vi "A170316-11-Main-large.vi"() -> ()   [LabVIEW 2020]
uses:
  System.Windows.Forms
  Database/Global1.vi
  Global_Variable/A170316-11.vi
  Global_Variable/Global.vi
  <userlib>/_MGI/Menu Building/MenuItemStatusChange/MGI_MenuItemStatusChange.lvclass
panel:
  out "提示信息 2":string
  out "ECU前序显示字":string
  out "电机前序显示字":string
  out "ECU装配\n前序状态":bool
  out "电机装配\n前序状态":bool
  out "电机码":string
  out "电机工位管柱码":string
  out "控制器码":string
  out "ECU自动":bool
  out "电机安装数量":u32
  out "ECU结果显示":string
  out "电机结果显示":string
  in  "质量报警":bool caption="布尔"
  in  "设备缺料":bool caption="布尔"
  in  "设备故障":bool caption="布尔"
  in  "设备离线":bool caption="布尔"
  in  "设备正常":bool caption="布尔"
  in  "菜单":refnum<k24>(container)
  out "检测结果":bool
  in  "批次信息":string[][](table)
  out "提示信息":string
  out "错误":bool
  out "时间字符串":string
  out "日期字符串":string
  out "电机自动":bool
  out "userStatus":string caption="用户状态"
  out "userName":string caption="用户名"
  out "安装支架数量":u32
  out "ECU工位管柱码":string
  out "connectionMode":string caption="联机类型"
  out "产品型号":string
  in  "更换产品":refnum<vi>
  # "电机ECU装配"
  # "控制器支架"
  # "安装支架(合装)"
  # "电机安装"
  # "安装支架检测结果"
  # "电机安装检测结果"
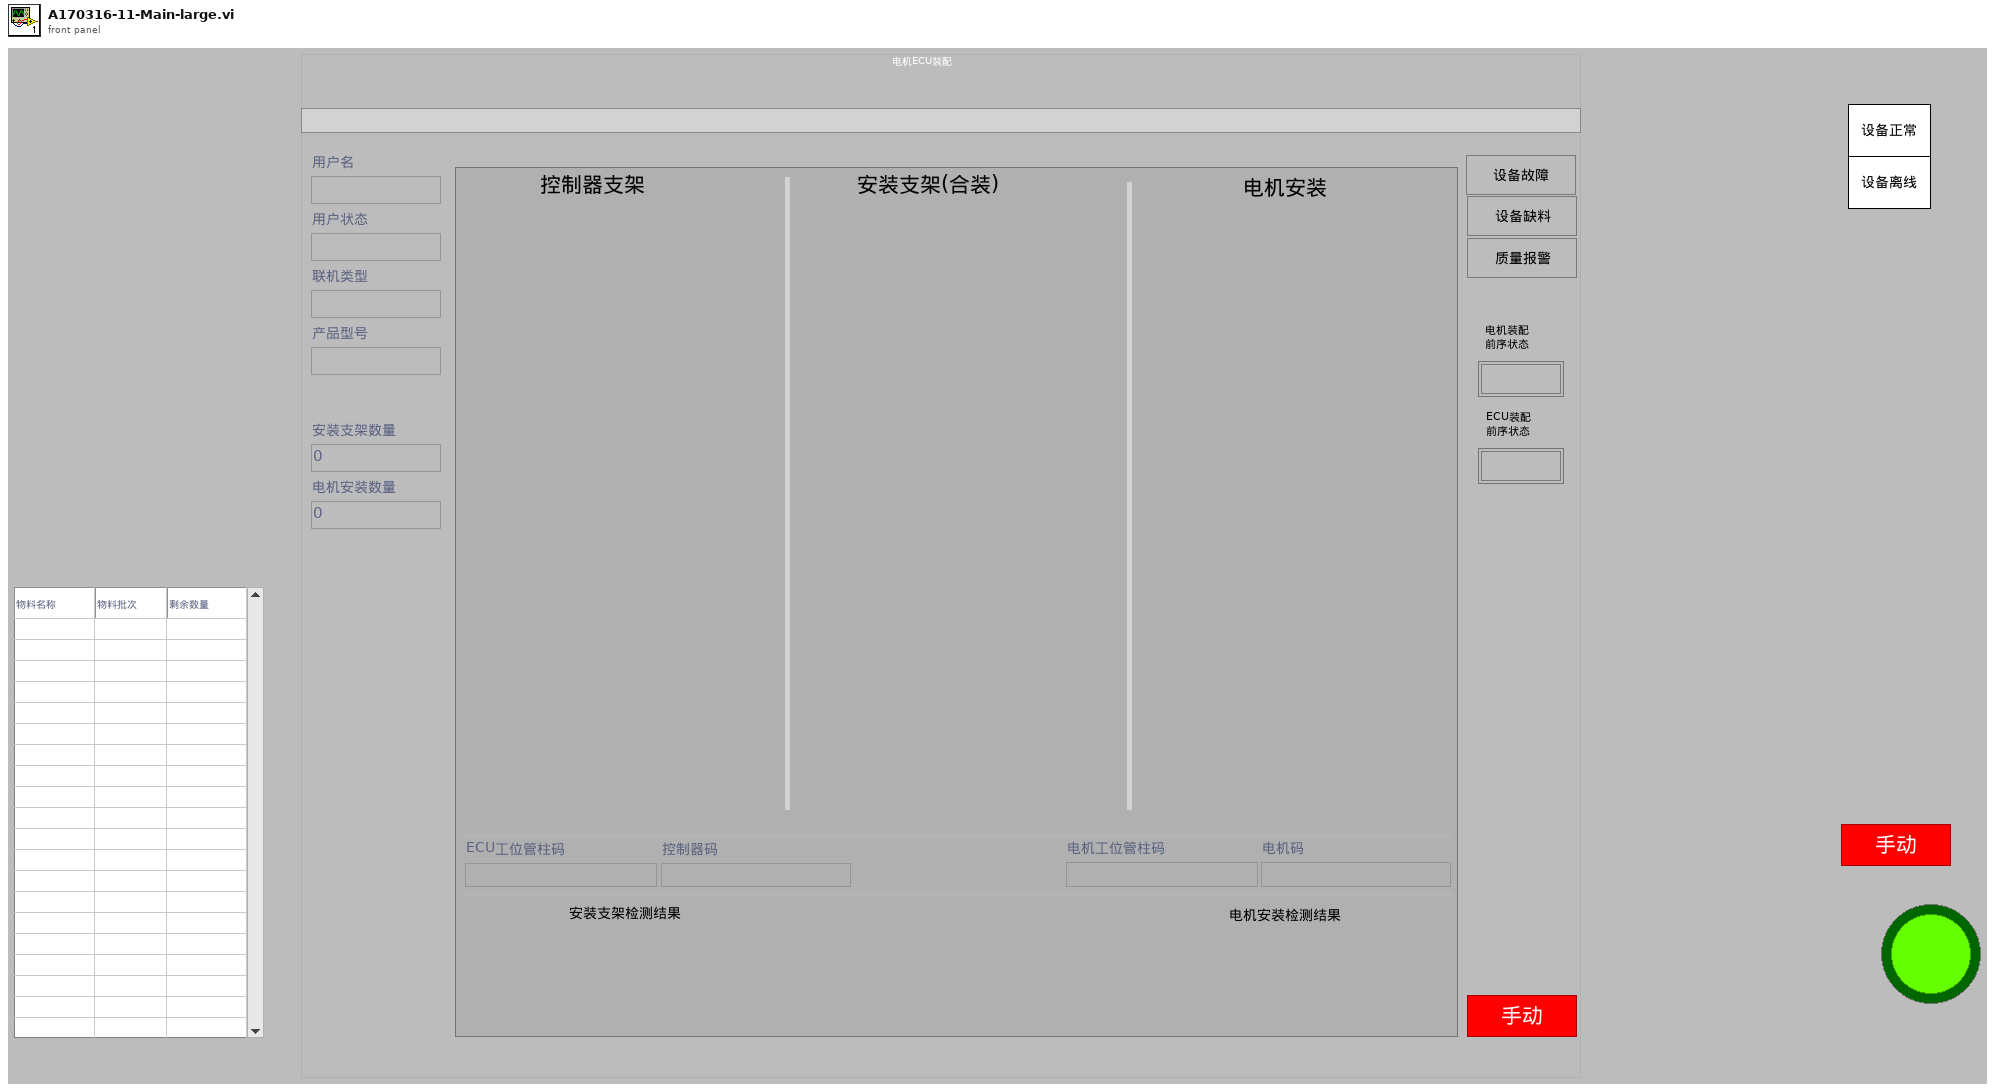
[diagram p1: front panel]
types:
  T1 = enum32{"Invalid", "Standard", "Closed", "Hidden", "Minimized", "Maximized"}
  T2 = enum32{"invalid app kind", "Development System", "Run Time System", "Student Edition", "Embedded LabVIEW", "Evaluation", "Custom"}
  T3 = cluster{"Core":cluster{"Current VI Reference":refnum<vi>, "Close Panel on Exit?":bool}, "Your Boolean data":bool, "Your string data":string}
  T4 = cluster{"Current VI Reference":refnum<vi>, "Close Panel on Exit?":bool}
  T5 = cluster{"用户编号":string, "用户名":string, "用户密码(密文)":string, "用户权限":string}
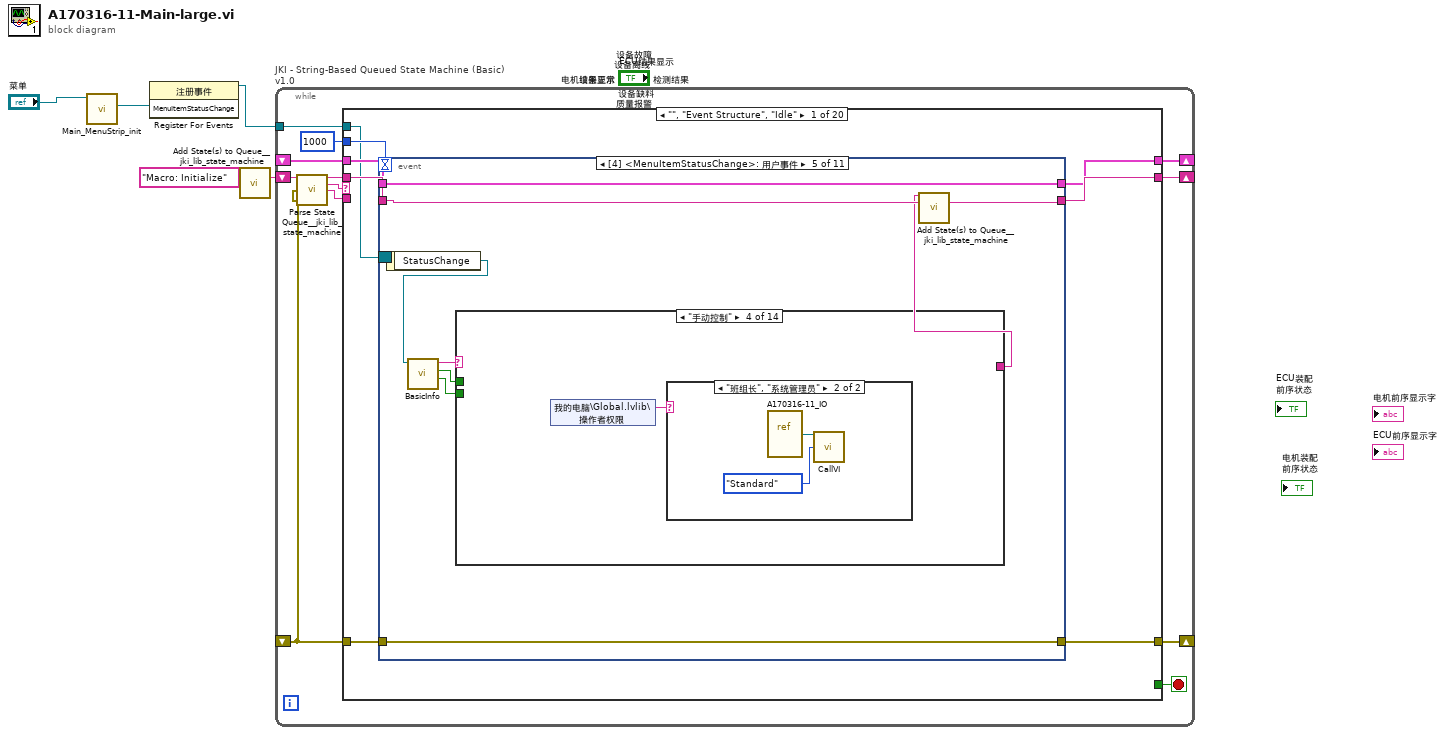
[diagram p0: block diagram]
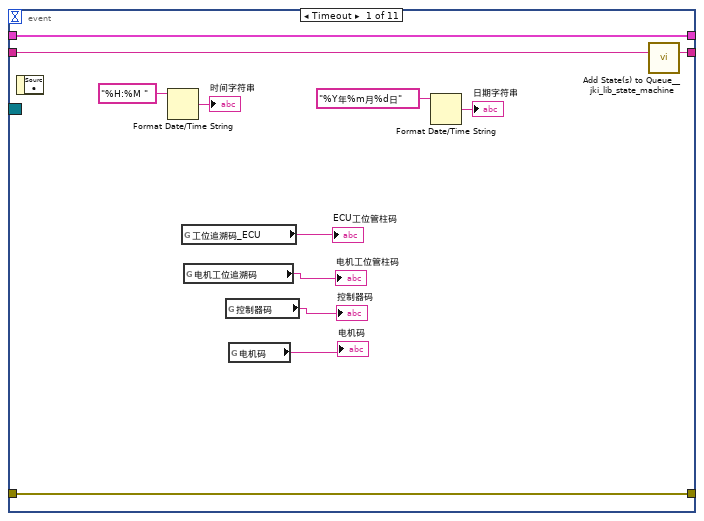
[diagram p2: hidden frame]
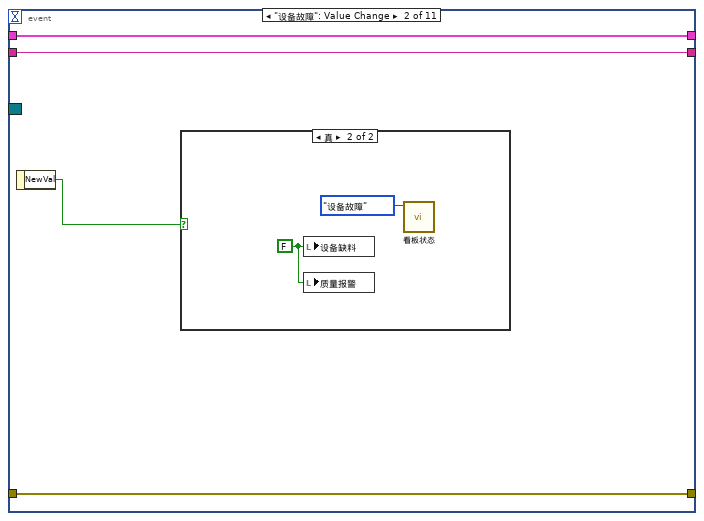
[diagram p3: hidden frame]
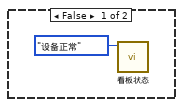
[diagram p4: hidden frame]
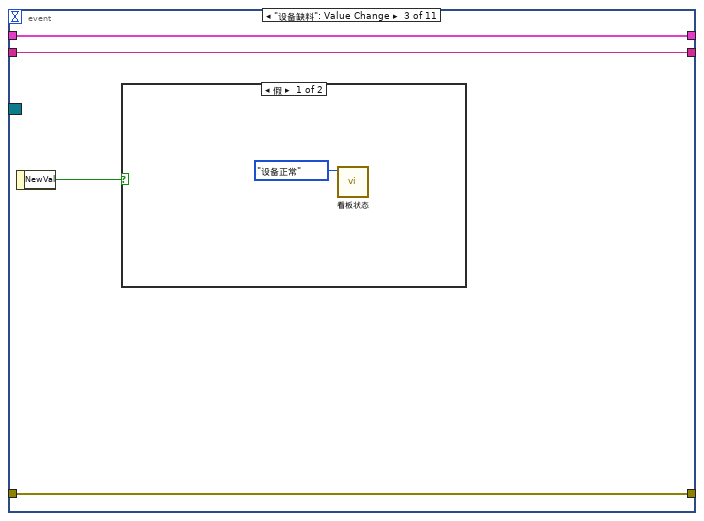
[diagram p5: hidden frame]
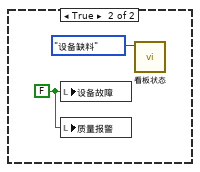
[diagram p6: hidden frame]
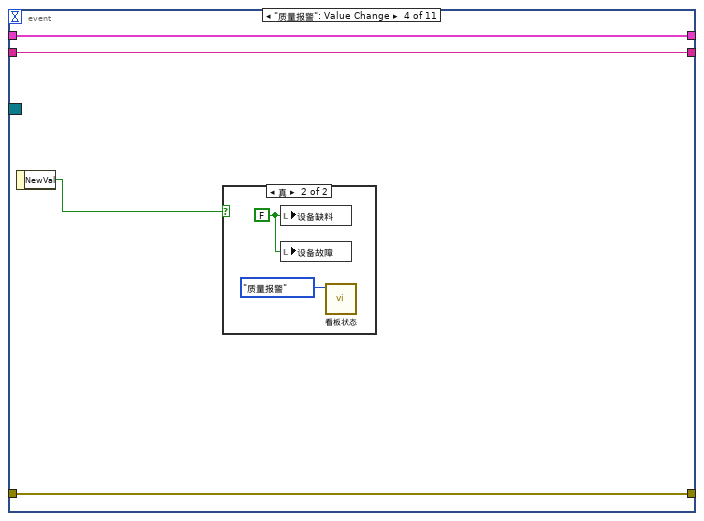
[diagram p7: hidden frame]
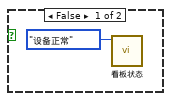
[diagram p8: hidden frame]
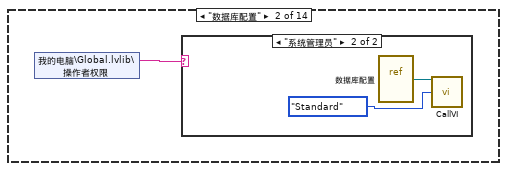
[diagram p10: hidden frame]
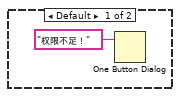
[diagram p11: hidden frame]
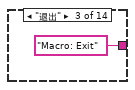
[diagram p12: hidden frame]
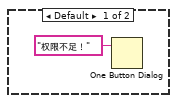
[diagram p13: hidden frame]
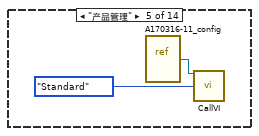
[diagram p14: hidden frame]
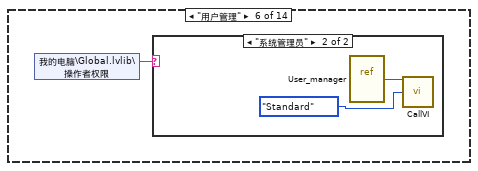
[diagram p15: hidden frame]
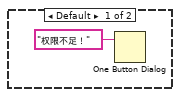
[diagram p16: hidden frame]
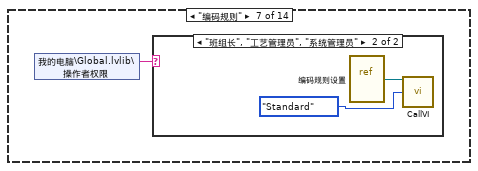
[diagram p17: hidden frame]
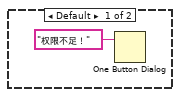
[diagram p18: hidden frame]
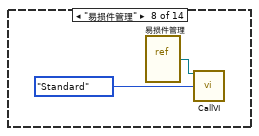
[diagram p19: hidden frame]
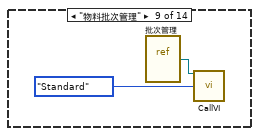
[diagram p20: hidden frame]
diagram:
  n1 = call "Main_MenuStrip_init.vi"("MenuStrip"="菜单") -> ("MenuItemStatusChange"=w2:refnum<user-event>)  [unwired: 9 in, 1 out]
  n2 = register-events(w2) -> (reference out=w1:refnum<event-registration>)  [unwired: 2 in, 1 out]
  n3 = call <vilib>:"Add State(s) to Queue__jki_lib_state_machine.vi"("State(s) in (\"\")"="Macro: Initialize") -> ("States Out"=w5:string)  [unwired: 14 in]
  n4 = while "JKI - String-Based Queued State Machine (Basic) v1.0" {
    shift-right: [w10] -> _
    shift-left: _ -> [w9]
    shift-right: [w13] -> _
    shift-left: _ -> [w7]
    shift-right: [w12] -> _
    shift-left: w5 -> [w14]
    tunnel: w1 -> [w6]
    stop <- w11 stop-if-true
    n5 = call <vilib>:"Parse State Queue__jki_lib_state_machine.vi"("State Queue"=w14, "Error In (no error)"=w7) -> ("Remaining States"=w16:string, "Current State"=w17:string, "Arguments"=w15:string)  [unwired: 11 in]
    n6 = case shown="\"\", \"Event Structure\", \"Idle\"" w17 {
      selector: w17 -> [_ _ w222 _ _ _ _ _ _ _ _ _ _ _ _ _ _ _ _ _]
      tunnel: w16 -> [w25 w221 w226 w244 w250 w255 w259 w266 w272 w276 w293 w319 w377 w388 w414 w419 w434 w438 w442 w446]
      tunnel: w15 -> [_ _ _ _ _ _ _ _ _ _ _ _ w372 w382 _ _ _ _ _ _]
      tunnel: w9 -> [w23 w218 w224 w235 w247 w253 w256 _ w267 w273 w291 w317 w375 w384 w411 w416 w431 w435 w439 w443]
      tunnel: [w22 w219 w228 w241 errorcluster {"status"=FALSE, "code"=0, "source"=""} ("error out") w252 w257 w263 w268 w274 w290 w316 w373 w385 w412 w417 w432 w436 w440 w444] -> w13
      tunnel: w7 -> [w21 w219 w227 w241 w246 w252 w257 w263 w269 w274 _ w316 w374 w386 w412 w417 w432 w436 w440 w444]
      tunnel: [w24 w220 w225 w243 w249 w254 w258 w265 w271 w275 w292 w318 w376 w387 w413 w418 w433 w437 w441 w445] -> w12
      tunnel: [_ _ _ _ _ TRUE _ _ _ _ _ _ _ _ _ _ _ _ _ _] -> w11
      tunnel: [w20 w218 w224 w242 w247 w253 w256 w264 w267 w273 w291 w317 w375 w384 w411 w416 w431 w435 w439 w443] -> w10
      tunnel: 1000 ("Timeout") -> [w19 _ _ _ _ _ _ _ _ _ _ _ _ _ _ _ _ _ _ _]
      tunnel: w6 -> [w18 _ _ _ _ _ _ _ _ _ _ _ _ _ _ _ _ _ _ _]
      frame "", "Event Structure", "Idle" {
        n7 = event shown="[4] <MenuItemStatusChange>: 用户事件" {
          selector: w18 -> [_ _ _ _ _ _ _ _ _ _ _]
          dyn-events: _ -> [_ _ _ _ _ _ _ _ _ _ _]
          timeout: w19 -> [_ _ _ _ _ _ _ _ _ _ _]
          tunnel: w25 -> [w37 w40 w47 w54 w62 w112 w162 w168 w202 w211 w214]
          tunnel: [w36 w40 w47 w54 w61 w110 w163 w168 w202 w210 w215] -> w24
          tunnel: w23 -> [w34 w41 w48 w55 w63 w111 w164 w169 w203 w208 w217]
          tunnel: [w35 w39 w46 w53 w59 w113 w161 w167 w201 w209 w216] -> w22
          tunnel: w21 -> [w35 w39 w46 w53 w59 w113 w161 w167 w201 w209 w216]
          tunnel: [w34 w41 w48 w55 w63 w111 w164 w169 w203 w208 w217] -> w20
          event Timeout {
            n8 = event-data() -> ()  [unwired: 1 in, 1 out]
            n9 = Format Date/Time String(time format string (%c)="%H:%M ") -> (date/time string=→"时间字符串":string)  [unwired: 2 in]
            n10 = global read "Global1.vi" "工位追溯码_ECU"() -> (→"ECU工位管柱码":string)
            n11 = global read "Global1.vi" "电机工位追溯码"() -> (→"电机工位管柱码":string)
            n12 = global read "Global1.vi" "控制器码"() -> (→"控制器码":string)
            n13 = global read "Global1.vi" "电机码"() -> (→"电机码":string)
            n14 = Format Date/Time String(time format string (%c)="%Y年%m月%d日") -> (date/time string=→"日期字符串":string)  [unwired: 2 in]
            n15 = call <vilib>:"Add State(s) to Queue__jki_lib_state_machine.vi"("State(s) in (\"\")"=w37) -> ("States Out"=w36:string)  [unwired: 14 in]
          }
          event "设备故障": Value Change {
            n16 = event-data() -> ("NewVal"=w38:bool)  [unwired: 1 in]
            n17 = case shown="真" w38 {
              frame False {
                n18 = call "看板状态.vi"("设备状态"=enum16{"设备离线", "设备正常", "设备缺料", "设备故障", "质量报警"}."设备正常") -> ()  [unwired: 10 in, 1 out]
              }
              frame True {
                w43 = FALSE ("质量报警")
                n19 = local write "设备缺料"(w43) -> ()
                n20 = local write "质量报警"(w43) -> ()
                n21 = call "看板状态.vi"("设备状态"=enum16{"设备离线", "设备正常", "设备缺料", "设备故障", "质量报警"}."设备故障") -> ()  [unwired: 10 in, 1 out]
              }
            }
          }
          event "设备缺料": Value Change {
            n22 = event-data() -> ("NewVal"=w45:bool)  [unwired: 1 in]
            n23 = case shown="假" w45 {
              frame False {
                n24 = call "看板状态.vi"("设备状态"=enum16{"设备离线", "设备正常", "设备缺料", "设备故障", "质量报警"}."设备正常") -> ()  [unwired: 10 in, 1 out]
              }
              frame True {
                w50 = FALSE ("质量报警")
                n25 = local write "设备故障"(w50) -> ()
                n26 = local write "质量报警"(w50) -> ()
                n27 = call "看板状态.vi"("设备状态"=enum16{"设备离线", "设备正常", "设备缺料", "设备故障", "质量报警"}."设备缺料") -> ()  [unwired: 10 in, 1 out]
              }
            }
          }
          event "质量报警": Value Change {
            n28 = event-data() -> ("NewVal"=w52:bool)  [unwired: 1 in]
            n29 = case shown="真" w52 {
              frame False {
                n30 = call "看板状态.vi"("设备状态"=enum16{"设备离线", "设备正常", "设备缺料", "设备故障", "质量报警"}."设备正常") -> ()  [unwired: 10 in, 1 out]
              }
              frame True {
                w57 = FALSE ("质量报警")
                n31 = local write "设备缺料"(w57) -> ()
                n32 = local write "设备故障"(w57) -> ()
                n33 = call "看板状态.vi"("设备状态"=enum16{"设备离线", "设备正常", "设备缺料", "设备故障", "质量报警"}."质量报警") -> ()  [unwired: 10 in, 1 out]
              }
            }
          }
          event User Event {
            n34 = event-data() -> ("StatusChange"=w64:refnum<class "MGI_MenuItemStatusChange.lvclass">)  [unwired: 1 in]
            n35 = call <userlib>:"BasicInfo.vi"("MGI_MenuItemStatusChange in"=w64) -> ("Enabled?"=w67:bool, "Checked?"=w66:bool, "Tag"=w65:string)  [unwired: 7 in, 1 out]
            n36 = case shown="\"手动控制\"" w65 {
              tunnel: w66 -> [_ _ _ _ _ _ _ _ _ _ _ _ _ _]
              tunnel: w67 -> [_ _ _ _ _ _ _ _ _ _ _ _ _ _]
              tunnel: [_ _ "Macro: Exit" _ _ _ _ _ _ _ _ _ _ _] -> w60
              frame Default {
              }
              frame "数据库配置" {
                n37 = shared-variable "我的电脑\\Global.lvlib\\操作者权限"() -> (w68:string)  [unwired: 1 in, 1 out]
                n38 = case shown="\"系统管理员\"" w68 {
                  frame Default {
                    n39 = One Button Dialog(message="权限不足！" ("消息")) -> ()  [unwired: 1 in, 1 out]
                  }
                  frame "系统管理员" {
                    n40 = vi-ref "数据库配置.vi"() -> (w71:refnum<vi>)
                    n41 = call "CallVI.vi"("VI引用"=w71, "状态"=T1."Standard") -> ()  [unwired: 11 in, 3 out]
                  }
                }
              }
              frame "退出" {
              }
              frame "手动控制" {
                n42 = shared-variable "我的电脑\\Global.lvlib\\操作者权限"() -> (w73:string)  [unwired: 1 in, 1 out]
                n43 = case shown="\"班组长\", \"系统管理员\"" w73 {
                  frame Default {
                    n44 = One Button Dialog(message="权限不足！" ("消息")) -> ()  [unwired: 1 in, 1 out]
                  }
                  frame "班组长", "系统管理员" {
                    n45 = vi-ref "A170316-11_IO.vi"() -> (w76:refnum<vi>)
                    n46 = call "CallVI.vi"("VI引用"=w76, "状态"=T1."Standard") -> ()  [unwired: 11 in, 3 out]
                  }
                }
              }
              frame "产品管理" {
                n47 = vi-ref "A170316-11_config.vi"() -> (w78:refnum<vi>)
                n48 = call "CallVI.vi"("VI引用"=w78, "状态"=T1."Standard") -> ()  [unwired: 11 in, 3 out]
              }
              frame "用户管理" {
                n49 = shared-variable "我的电脑\\Global.lvlib\\操作者权限"() -> (w79:string)  [unwired: 1 in, 1 out]
                n50 = case shown="\"系统管理员\"" w79 {
                  frame Default {
                    n51 = One Button Dialog(message="权限不足！" ("消息")) -> ()  [unwired: 1 in, 1 out]
                  }
                  frame "系统管理员" {
                    n52 = vi-ref "User_manager.vi"() -> (w82:refnum<vi>)
                    n53 = call "CallVI.vi"("VI引用"=w82, "状态"=T1."Standard") -> ()  [unwired: 11 in, 3 out]
                  }
                }
              }
              frame "编码规则" {
                n54 = shared-variable "我的电脑\\Global.lvlib\\操作者权限"() -> (w83:string)  [unwired: 1 in, 1 out]
                n55 = case shown="\"班组长\", \"工艺管理员\", \"系统管理员\"" w83 {
                  frame Default {
                    n56 = One Button Dialog(message="权限不足！" ("消息")) -> ()  [unwired: 1 in, 1 out]
                  }
                  frame "班组长", "工艺管理员", "系统管理员" {
                    n57 = vi-ref "编码规则设置.vi"() -> (w86:refnum<vi>)
                    n58 = call "CallVI.vi"("VI引用"=w86, "状态"=T1."Standard") -> ()  [unwired: 11 in, 3 out]
                  }
                }
              }
              frame "易损件管理" {
                n59 = vi-ref "易损件管理.vi"() -> (w88:refnum<vi>)
                n60 = call "CallVI.vi"("VI引用"=w88, "状态"=T1."Standard") -> ()  [unwired: 11 in, 3 out]
              }
              frame "物料批次管理" {
                n61 = vi-ref "批次管理.vi"() -> (w90:refnum<vi>)
                n62 = call "CallVI.vi"("VI引用"=w90, "状态"=T1."Standard") -> ()  [unwired: 11 in, 3 out]
              }
              frame "设备管理" {
                n63 = vi-ref "注册设备.vi"() -> (w92:refnum<vi>)
                n64 = call "CallVI.vi"("VI引用"=w92, "状态"=T1."Standard") -> ()  [unwired: 11 in, 3 out]
              }
              frame "报表" {
                n65 = call "文件对话框2"("start path"=path "D:/report", "prompt"="打开报表", "pattern (all files)"="*.doc;*.docx", "pattern label"="Word 文档") -> ("selected path"=w93:path, "error out"=w94:errorcluster)  [unwired: 8 in, 2 out]
                n66 = case shown="无错误" w94 {
                  selector: w94 -> [w100 w102]
                  tunnel: w93 -> [w101 _]
                  frame No Error {
                    w99 = 1 items=["Normal", "Maximize", "Minimize"] ("cpubbs_WindowState")
                    n67 = call "Open_Word.vi"("File Path"=w101, "cpubbs_WindowState"=w99, "错误输入（无错误）"=w100) -> ()  [unwired: 12 in, 1 out]
                  }
                  frame Error {
                    n68 = call <vilib>:"Clear Errors.vi"("error in (no error)"=w102) -> ()  [unwired: 5 in, 2 out]
                  }
                }
              }
              frame "报警信息" {
                n69 = vi-ref "报警信息.vi"() -> (w104:refnum<vi>)
                n70 = call "CallVI.vi"("VI引用"=w104, "状态"=T1."Standard") -> ()  [unwired: 11 in, 3 out]
              }
              frame "关于" {
                n71 = vi-ref "About.vi"() -> (w106:refnum<vi>)
                n72 = call "CallVI.vi"("VI引用"=w106, "状态"=T1."Standard") -> ()  [unwired: 11 in, 3 out]
              }
              frame "操作演示" {
                n73 = call <vilib>:"Application Directory.vi"() -> ("Application Directory"=w109:path)
                n74 = Build Path(base path=w109, name or relative path="操作演示" ("名称或相对路径")) -> (appended path=w108:path)
                n75 = call "自动播放ppt.vi"("路径"=w108) -> ()  [unwired: 10 in, 1 out]
              }
            }
            n76 = call <vilib>:"Add State(s) to Queue__jki_lib_state_machine.vi"("State(s) in Front (\"\")"=w60, "State(s) in (\"\")"=w62) -> ("States Out"=w61:string)  [unwired: 13 in]
          }
          event Menu Selection (User) {
            n77 = event-data() -> ("ItemTag"=w114:string)  [unwired: 1 in, 6 out]
            n78 = case shown="\"手动控制\"" w114 {
              frame "假", Default {
              }
              frame "数据库配置" {
                n79 = shared-variable "我的电脑\\Global.lvlib\\操作者权限"() -> (w115:string)  [unwired: 1 in, 1 out]
                n80 = case shown="\"系统管理员\"" w115 {
                  frame Default {
                    n81 = One Button Dialog(message="权限不足！" ("消息")) -> ()  [unwired: 1 in, 1 out]
                  }
                  frame "系统管理员" {
                    n82 = vi-ref "数据库配置.vi"() -> (w118:refnum<vi>)
                    n83 = call "CallVI.vi"("VI引用"=w118, "状态"=T1."Standard") -> ()  [unwired: 11 in, 3 out]
                  }
                }
              }
              frame "退出" {
                n84 = Quit LabVIEW() -> ()  [unwired: 1 in]
              }
              frame "手动控制" {
                n85 = shared-variable "我的电脑\\Global.lvlib\\操作者权限"() -> (w119:string)  [unwired: 1 in, 1 out]
                n86 = case shown="\"班组长\", \"系统管理员\"" w119 {
                  frame Default {
                    n87 = One Button Dialog(message="权限不足！" ("消息")) -> ()  [unwired: 1 in, 1 out]
                  }
                  frame "班组长", "系统管理员" {
                    n88 = vi-ref "A170316-11_IO.vi"() -> (w122:refnum<vi>)
                    n89 = call "CallVI.vi"("VI引用"=w122, "状态"=T1."Standard") -> ()  [unwired: 11 in, 3 out]
                  }
                }
              }
              frame "半自动控制" {
                n90 = disable-structure shown="启用" {
                  frame Disabled {
                    n91 = shared-variable "我的电脑\\Global.lvlib\\操作者权限"() -> (w123:string)  [unwired: 1 in, 1 out]
                    n92 = case shown="\"班组长\", \"系统管理员\"" w123 {
                      frame Default {
                        n93 = One Button Dialog(message="权限不足！" ("消息")) -> ()  [unwired: 1 in, 1 out]
                      }
                      frame "班组长", "系统管理员" {
                        n94 = call "CallVI.vi"("VI引用"=refnum<vi> refnum, "状态"=T1."Maximized") -> ()  [unwired: 11 in, 3 out]
                      }
                    }
                  }
                  frame Enabled {
                    n95 = One Button Dialog(message="当前设备不具备半自动功能！" ("消息")) -> ()  [unwired: 1 in, 1 out]
                  }
                }
              }
              frame "产品管理" {
                n96 = vi-ref "A170316-11_config.vi"() -> (w129:refnum<vi>)
                n97 = call "CallVI.vi"("VI引用"=w129, "状态"=T1."Standard") -> ()  [unwired: 11 in, 3 out]
              }
              frame "系统配置" {
              }
              frame "用户管理" {
                n98 = shared-variable "我的电脑\\Global.lvlib\\操作者权限"() -> (w130:string)  [unwired: 1 in, 1 out]
                n99 = case shown="\"系统管理员\"" w130 {
                  frame Default {
                    n100 = One Button Dialog(message="权限不足！" ("消息")) -> ()  [unwired: 1 in, 1 out]
                  }
                  frame "系统管理员" {
                    n101 = vi-ref "User_manager.vi"() -> (w133:refnum<vi>)
                    n102 = call "CallVI.vi"("VI引用"=w133, "状态"=T1."Standard") -> ()  [unwired: 11 in, 3 out]
                  }
                }
              }
              frame "编码规则" {
                n103 = shared-variable "我的电脑\\Global.lvlib\\操作者权限"() -> (w134:string)  [unwired: 1 in, 1 out]
                n104 = case shown="\"班组长\", \"工艺管理员\", \"系统管理员\"" w134 {
                  frame Default {
                    n105 = One Button Dialog(message="权限不足！" ("消息")) -> ()  [unwired: 1 in, 1 out]
                  }
                  frame "班组长", "工艺管理员", "系统管理员" {
                    n106 = vi-ref "编码规则设置.vi"() -> (w137:refnum<vi>)
                    n107 = call "CallVI.vi"("VI引用"=w137, "状态"=T1."Standard") -> ()  [unwired: 11 in, 3 out]
                  }
                }
              }
              frame "易损件管理" {
                n108 = vi-ref "易损件管理.vi"() -> (w139:refnum<vi>)
                n109 = call "CallVI.vi"("VI引用"=w139, "状态"=T1."Standard") -> ()  [unwired: 11 in, 3 out]
              }
              frame "物料批次管理" {
                n110 = vi-ref "批次管理.vi"() -> (w141:refnum<vi>)
                n111 = call "CallVI.vi"("VI引用"=w141, "状态"=T1."Standard") -> ()  [unwired: 11 in, 3 out]
              }
              frame "打开报表" {
                n112 = call "文件对话框"("start path"=path "D:/report", "prompt"="打开报表", "pattern (all files)"="*.doc;*.docx", "pattern label"="Word 文档") -> ("selected path"=w142:path, "error out"=w143:errorcluster)  [unwired: 8 in, 2 out]
                n113 = case shown="无错误" w143 {
                  selector: w143 -> [w149 w151]
                  tunnel: w142 -> [w150 _]
                  frame No Error {
                    w148 = 1 items=["Normal", "Maximize", "Minimize"] ("cpubbs_WindowState")
                    n114 = call "Open_Word.vi"("File Path"=w150, "cpubbs_WindowState"=w148, "错误输入（无错误）"=w149) -> ()  [unwired: 12 in, 1 out]
                  }
                  frame Error {
                    n115 = call <vilib>:"Clear Errors.vi"("error in (no error)"=w151) -> ()  [unwired: 5 in, 2 out]
                  }
                }
              }
              frame "报警信息" {
                n116 = vi-ref "报警信息.vi"() -> (w153:refnum<vi>)
                n117 = call "CallVI.vi"("VI引用"=w153, "状态"=T1."Standard") -> ()  [unwired: 11 in, 3 out]
              }
              frame "关于" {
                n118 = vi-ref "About.vi"() -> (w155:refnum<vi>)
                n119 = call "CallVI.vi"("VI引用"=w155, "状态"=T1."Standard") -> ()  [unwired: 11 in, 3 out]
              }
              frame "操作演示" {
                n120 = call <vilib>:"Application Directory.vi"() -> ("Application Directory"=w158:path)
                n121 = Build Path(base path=w158, name or relative path="操作演示" ("名称或相对路径")) -> (appended path=w157:path)
                n122 = call "自动播放ppt.vi"("路径"=w157) -> ()  [unwired: 10 in, 1 out]
              }
            }
            n123 = call <vilib>:"Add State(s) to Queue__jki_lib_state_machine.vi"("State(s) in (\"\")"=w112) -> ("States Out"=w110:string)  [unwired: 14 in]
          }
          event "错误": Mouse Down {
            n124 = event-data() -> ()  [unwired: 1 in, 8 out]
            n125 = vi-ref "报警信息.vi"() -> (w160:refnum<vi>)
            n126 = call "CallVI.vi"("VI引用"=w160, "状态"=T1."Standard") -> ()  [unwired: 11 in, 3 out]
            n127 = call <vilib>:"Add State(s) to Queue__jki_lib_state_machine.vi"("State(s) in (\"\")"=w162) -> ("States Out"=w163:string)  [unwired: 14 in]
          }
          event "电机自动": Mouse Down {
            n128 = event-data() -> ("CtlRef"=w166:refnum<vi>)  [unwired: 1 in, 7 out]
            n129 = property class="Bool (严格)"(reference=w166) -> ("Value"=w165:bool)  [unwired: 1 in, 2 out]
            n130 = case shown="真" w165 {
              frame False {
                n131 = shared-variable "我的电脑\\A17031611.lvlib\\设备状态3"() -> (w170:i16)  [unwired: 1 in, 1 out]
                n132 = case shown="5" w170 {
                  frame 0, Default {
                    n133 = call "浮动通知.vi"("通知内容"="请复位！") -> ()  [unwired: 11 in]
                  }
                  frame 5 {
                    n134 = vi-ref "A170316-11_Auto.vi"() -> (w172:refnum<vi>)
                    n135 = invoke class="VI" method="Ctrl Val.Set"(reference=w172, "Control Name"="STEP3" ("控件名"), "Value"="初始化" ("控件名")) -> ()  [unwired: 2 in, 5 out]
                    n136 = invoke class="VI" method="Ctrl Val.Set"(reference=w172, "Control Name"="STEP2" ("控件名"), "Value"="初始化" ("控件名")) -> (reference out=w180:refnum<vi>, error out=w179:errorcluster)  [unwired: 2 in, 3 out]
                    n137 = invoke class="VI" method="Ctrl Val.Set"(reference=w180, error in=w179, "Control Name"="STEP1" ("控件名"), "Value"="初始化" ("控件名")) -> ()  [unwired: 1 in, 5 out]
                  }
                }
              }
              frame True {
                n138 = global read "A170316-11.vi" "电机安装LED"() -> (w182:refnum<vi>[])
                n139 = global read "A170316-11.vi" "安装支架LED"() -> (w183:refnum<vi>[])
                n140 = global read "A170316-11.vi" "控制器支架LED"() -> (w181:refnum<vi>[])
                n141 = Two Button Dialog(message="自动程序运行中，\n是否切换为手动？" ("消息")) -> (T button?=w184:bool)  [unwired: 2 in]
                n142 = case shown="真" w184 {
                  tunnel: w183 -> [_ w194]
                  tunnel: w182 -> [_ w193]
                  tunnel: w181 -> [_ w192]
                  frame False {
                  }
                  frame True {
                    n143 = for {
                      tunnel: w194 -> [w199] mode=indexing
                      n144 = call "Colour.vi"("result"="", "colourRef"=w199) -> ()  [unwired: 9 in, 1 out]
                    }
                    n145 = vi-ref "A170316-11_Auto.vi"() -> (w191:refnum<vi>)
                    n146 = for {
                      tunnel: w192 -> [w195] mode=indexing
                      n147 = call "Colour.vi"("result"="", "colourRef"=w195) -> ()  [unwired: 9 in, 1 out]
                    }
                    n148 = invoke class="VI" method="Ctrl Val.Set"(reference=w191, "Control Name"="STEP3" ("控件名"), "Value"="手动" ("控件名")) -> (reference out=w188:refnum<vi>)  [unwired: 2 in, 4 out]
                    n149 = for {
                      tunnel: w193 -> [w197] mode=indexing
                      n150 = call "Colour.vi"("result"="", "colourRef"=w197) -> ()  [unwired: 9 in, 1 out]
                    }
                    n151 = invoke class="VI" method="Ctrl Val.Set"(reference=w188, "Control Name"="STEP2" ("控件名"), "Value"="手动" ("控件名")) -> ()  [unwired: 2 in, 5 out]
                  }
                }
              }
            }
          }
          event "ECU自动": Mouse Down {
            n152 = event-data() -> ()  [unwired: 1 in, 8 out]
          }
          event Panel Close? {
            n153 = event-data() -> ()  [unwired: 1 in, 1 out]
            n154 = control-ref of="本VI"() -> (w204:refnum<vi>)
            n155 = invoke class="VI" method="FP.Close"(reference=w204) -> ()  [unwired: 2 in, 3 out]
            n156 = global write "Global.vi" "程序关闭"(TRUE ("程序关闭")) -> ()
            n157 = event-data("Discard?"=TRUE) -> ()  [unwired: 1 in, 1 out]
            n158 = call <vilib>:"Add State(s) to Queue__jki_lib_state_machine.vi"("State(s) in Front (\"\")"="Macro: Exit", "State(s) in (\"\")"=w211) -> ("States Out"=w210:string)  [unwired: 13 in]
          }
          event "更换产品": Value Change {
            n159 = event-data() -> ("NewVal"=w213:refnum<vi>)  [unwired: 1 in, 5 out]
            n160 = control-ref of="ECU工位"() -> (w212:refnum<vi>)
            n161 = call "Call_SubPanal.vi"("VI引用句柄"=w213, "SubPnl引用句柄"=w212) -> ()  [unwired: 9 in, 1 out]
            n162 = call <vilib>:"Add State(s) to Queue__jki_lib_state_machine.vi"("State(s) in (\"\")"=w214) -> ("States Out"=w215:string)  [unwired: 14 in]
          }
        }
      }
      frame "---------- Core ----------" {
        n163 = call <vilib>:"Add State(s) to Queue__jki_lib_state_machine.vi"("State(s) in (\"\")"=w221) -> ("States Out"=w220:string)  [unwired: 14 in]
      }
      frame Default {
        w231 = 42 items=["No error", "Argument error", "Memory is full", "Out of zone", "End of file", "File already open", "Generic file I/O error", "File not found", "File permission error", "Disk is full", "Duplicate path", "Too many files open", "System feature not enabled", "Resource file not found", "Cannot add resource", "Resource not found", "Image not found", "Image memory error", "Pen does not exist", "Config type invalid", "Config token not found", "Config parse error", "Config memory error", "Bad external code format", "Bad external code offset", "External code not present", "Null window", "Destroy window error", "Null menu", "Print aborted", "Bad print record", "Print driver error", "Windows error during printing", "Memory error during printing", "Print dialog error", "Generic print error", "Invalid device refnum", "Device not found", "Device parameter error", "Device unit error", "Cannot open device", "Device call aborted", "Generic error", "Cancelled by user", "Object ID too low", "Object ID too high", "Object not in heap", "Unknown heap", "Unknown object (invalid DefProc)", "Unknown object (DefProc not in table)", "Message out of range", "Invalid (null) method", "Unknown message", "Manager call not supported", "Bad address", "Network operation in progress", "Network operation timed out", "Connection is busy", "Network attribute not supported", "Network error", "Address in use", "System out of memory", "Connection aborted", "Connection refused", "Not connected", "Already connected", "Connection closed", "Initialization error (interapplication manager)", "Bad occurrence", "Wait on unbound occurrence handler", "Occurrence queue overflow", "Datalog type conflict", "Unused", "Unrecognized type (interapplication manager)", "Memory corrupt", "Failed to make temporary DLL", "Old CIN version", "Drag socket not found", "Failed to load drop-object", "Failed to register OLE object", "Failed to release OLE object", "Format specifier type mismatch", "Unknown format specifier", "Too few format specifiers", "Too many format specifiers", "Scan failed", "Newer CIN version", "Error converting to variant", "Runtime menu error", "Password tampered", "Variant attribute not found", "Incompatible variant data type", "Event data is not available", "Event Store is not present", "Occurrence is not found", "Event Queue is not created", "Event info is not available", "Refnum passed is NULL", "Error retrieving Class GUID", "Error retrieving CoClass GUID", "Error retrieving TypeLib GUID.", "Bad built application magic bytes.", "Specific driver is different from the specific driver associated with the Logical Name.", "There is no session opened to the class driver.", "Max Error", "MAX - Error with config objects", "MAX - Error loading configuration", "MAX - Group not supported"]
        # "Current State"
        n164 = Format Into String(format string="Software Exception: Unhandled State \"%s\"." ("message"), error in=w227, w222) -> (resulting string=w230:string, error out=w229:errorcluster)  [unwired: 1 in]
        n165 = call <vilib>:"Error Cluster From Error Code.vi"("show call chain? (False)"=TRUE, "error in (no error)"=w229, "error message (\"\")"=w230, "error code (0)"=w231) -> ("error out"=w228:errorcluster)  [unwired: 5 in]
        n166 = call <vilib>:"Add State(s) to Queue__jki_lib_state_machine.vi"("State(s) in (\"\")"=w226) -> ("States Out"=w225:string)  [unwired: 14 in]
      }
      frame "Initialize Core Data" {
        # "originally closed?"
        # "exe?"
        n167 = property class="VI"() -> ("Front Panel.Open"=w240:bool)  [unwired: 2 in, 2 out]
        n168 = property class="App"() -> ("App.Kind"=w239:T2)  [unwired: 2 in, 2 out]
        n169 = control-ref of="Current VI Reference"() -> (w233:refnum<vi>)
        n170 = Not(x=w240) -> (.not. x?=w237:bool)
        n171 = Equal?(x=w239, y=T2."Run Time System" ("Application:Kind")) -> (x = y?=w236:bool)
        n172 = Or(x=w237, y=w236) -> (x .or. y?=w234:bool)
        n173 = Bundle By Name(cluster=w235, "Core.Current VI Reference"=w233, "Core.Close Panel on Exit?"=w234) -> (w242:T3)
        n174 = call <vilib>:"Add State(s) to Queue__jki_lib_state_machine.vi"("State(s) in (\"\")"=w244) -> ("States Out"=w243:string)  [unwired: 14 in]
      }
      frame "Error Handler" {
        n175 = call <vilib>:"General Error Handler.vi"("error in (no error)"=w246) -> ()  [unwired: 10 in, 5 out]
        n176 = call <vilib>:"Add State(s) to Queue__jki_lib_state_machine.vi"("State(s) in Front (\"\")"="/* Post Error States", "State(s) in (\"\")"=w250) -> ("States Out"=w249:string)  [unwired: 13 in]
      }
      frame "Exit" {
        n177 = call <vilib>:"Add State(s) to Queue__jki_lib_state_machine.vi"("State(s) in (\"\")"=w255) -> ("States Out"=w254:string)  [unwired: 14 in]
      }
      frame "---------- Data ----------" {
        n178 = call <vilib>:"Add State(s) to Queue__jki_lib_state_machine.vi"("State(s) in (\"\")"=w259) -> ("States Out"=w258:string)  [unwired: 14 in]
      }
      frame "Data: Initialize" {
        w260 = T4 {"Current VI Reference"=refnum, "Close Panel on Exit?"=FALSE}  # Core
        w262 = TRUE  # Your Boolean data
        w261 = ""  # Your string data
        n179 = Bundle("Core"=w260, "Your Boolean data"=w262, "Your string data"=w261) -> (w264:T3)  [unwired: 1 in]
        n180 = call <vilib>:"Add State(s) to Queue__jki_lib_state_machine.vi"("State(s) in (\"\")"=w266) -> ("States Out"=w265:string)  [unwired: 14 in]
      }
      frame "Data: Cleanup" {
        n181 = Unbundle By Name(w267) -> ("Core.Current VI Reference"=w270:refnum<vi>)
        n182 = Close Reference(reference=w270, error in (no error)=w269) -> (error out=w268:errorcluster)
        n183 = call <vilib>:"Add State(s) to Queue__jki_lib_state_machine.vi"("State(s) in (\"\")"=w272) -> ("States Out"=w271:string)  [unwired: 14 in]
      }
      frame "---------- UI ----------" {
        # "Do not put any code in this frame.\n(It is a separator no-op. You can make a copy of this frame to create a new UI frame)"
        n184 = call <vilib>:"Add State(s) to Queue__jki_lib_state_machine.vi"("State(s) in (\"\")"=w276) -> ("States Out"=w275:string)  [unwired: 14 in]
      }
      frame "UI: Initialize" {
        n185 = vi-ref "A170316-11_Auto.vi"() -> (w284:refnum<vi>)
        n186 = disable-structure shown="禁用" {
          frame Disabled {
            n187 = vi-ref "A170316-11_Auto -ECU.vi"() -> (w294:refnum<vi>)
            n188 = property class="VI"(reference=w294) -> (reference out=w299:refnum<vi>, error out=w301:errorcluster, "FP.State"=w298:T1)  [unwired: 1 in]
            n189 = case shown="\"Standard\"" w298 {
              tunnel: w299 -> [w305 w309]
              tunnel: [w305 w306] -> w303
              tunnel: [w304 w307] -> w300
              tunnel: w301 -> [w304 w308]
              frame "Invalid", "Closed", Default {
              }
              frame "Standard" {
                n190 = invoke class="VI" method="FP.Close"(reference=w309, error in=w308) -> (reference out=w306:refnum<vi>, error out=w307:errorcluster)  [unwired: 1 in, 1 out]
              }
            }
            n191 = invoke class="SubPnl" method="Insert VI"(error in=w300, "VI Ref"=w303) -> (reference=w295:refnum<vi>, error out=w302:errorcluster)  [unwired: 1 in, 3 out]
            n192 = invoke class="VI" method="Run VI"(reference=w303, error in=w302, "Wait until done"=FALSE ("结束前等待"), "Auto Dispose Ref"=TRUE ("自动销毁引用")) -> ()  [unwired: 1 in, 5 out]
          }
          frame Enabled {
          }
        }
        n193 = property class="VI"(reference=w284) -> (reference out=w282:refnum<vi>, error out=w279:errorcluster, "FP.State"=w283:T1)  [unwired: 1 in]
        n194 = control-ref of="ECU工位"() -> (w281:refnum<vi>)
        n195 = case shown="\"Standard\"" w283 {
          tunnel: w282 -> [w311 w315]
          tunnel: [w311 w312] -> w277
          tunnel: [w310 w313] -> w280
          tunnel: w279 -> [w310 w314]
          frame "Invalid", "Closed", Default {
          }
          frame "Standard" {
            n196 = invoke class="VI" method="FP.Close"(reference=w315, error in=w314) -> (reference out=w312:refnum<vi>, error out=w313:errorcluster)  [unwired: 1 in, 1 out]
          }
        }
        n197 = invoke class="SubPnl" method="Insert VI"(reference=w281, error in=w280, "VI Ref"=w277) -> (error out=w278:errorcluster)  [unwired: 1 in, 3 out]
        n198 = invoke class="VI" method="Run VI"(reference=w277, error in=w278, "Wait until done"=FALSE ("结束前等待"), "Auto Dispose Ref"=TRUE ("自动销毁引用")) -> (error out=w287:errorcluster)  [unwired: 1 in, 4 out]
        n199 = call "窗口自动调整.vi"("error in (no error)"=w287, "max？"=TRUE, "border spacing (2 px)"=0) -> ("error out"=w290:errorcluster)  [unwired: 3 in, 1 out]
        n200 = call <vilib>:"Add State(s) to Queue__jki_lib_state_machine.vi"("State(s) in (\"\")"=w293) -> ("States Out"=w292:string)  [unwired: 14 in]
      }
      frame "UI: Init" {
        n201 = stacked-sequence {
          frame #0 {
            w328 = u32 0 ("合格数量")
            w327 = "" ("输出轴码")
            n202 = global read "Global1.vi" "电机上序状态"() -> (w324:refnum<vi>)
            n203 = shared-variable "我的电脑\\Global.lvlib\\联机模式"() -> (w330:i16)  [unwired: 1 in, 1 out]
            n204 = global read "Global1.vi" "ECU上序状态"() -> (w326:refnum<vi>)
            n205 = case shown="1" w330 {
              tunnel: ["联网" ("connectionMode") "单机" ("connectionMode")] -> w331
              frame 1 {
              }
              frame 0, Default {
              }
            }
            "connectionMode" <- w331
            n206 = call "Colour.vi"("result"="", "colourRef"=w324) -> ()  [unwired: 9 in, 1 out]
            n207 = call "Colour.vi"("result"="", "colourRef"=w326) -> ()  [unwired: 9 in, 1 out]
            n208 = global read "Global1.vi" "用户信息"() -> (w322:T5)
            n209 = Unbundle By Name(w322) -> ("用户名"=→"userName":string, "用户权限"=→"userStatus":string)
            n210 = global write "Global1.vi" "电机工位追溯码"(w327) -> ()
            n211 = global write "Global1.vi" "工位追溯码_ECU"(w327) -> ()
            n212 = global write "Global1.vi" "电机码"(w327) -> ()
            n213 = global write "Global1.vi" "控制器码"(w327) -> ()
            "安装支架数量" <- w328
            "产品型号" <- "" ("productsName")
            "电机安装数量" <- w328
          }
          frame #1 {
            n214 = control-ref of="电机自动"() -> (w345:refnum<vi>)
            n215 = control-ref of="ECU自动"() -> (w339:refnum<vi>)
            n216 = control-ref of="更换产品"() -> (w343:refnum<vi>)
            n217 = global write "Global.vi" "电机程序自动"(w345) -> ()
            n218 = global write "Global.vi" "ECU自动"(w339) -> ()
            n219 = control-ref of="批次信息"() -> (w347:refnum<vi>)
            n220 = control-ref of="ECU前序显示字"() -> (w336:refnum<vi>)
            n221 = control-ref of="电机前序显示字"() -> (w335:refnum<vi>)
            n222 = global write "Global.vi" "更换产品"(w343) -> ()
            n223 = global write "Global.vi" "批次"(w347) -> ()
            n224 = global write "Global.vi" "ECU前序显示字"(w336) -> ()
            n225 = global write "Global.vi" "电机前序显示字"(w335) -> ()
            n226 = control-ref of="提示信息 2"() -> (w334:refnum<vi>)
            n227 = control-ref of="错误"() -> (w346:refnum<vi>)
            n228 = global write "Global.vi" "报警图标"(w346) -> ()
            n229 = global write "Global.vi" "提示信息 2"(w334) -> ()
            n230 = control-ref of="电机结果显示"() -> (w340:refnum<vi>)
            n231 = control-ref of="ECU结果显示"() -> (w337:refnum<vi>)
            n232 = control-ref of="提示信息"() -> (w344:refnum<vi>)
            n233 = control-ref of="电机安装数量"() -> (w338:refnum<vi>)
            n234 = control-ref of="安装支架数量"() -> (w342:refnum<vi>)
            n235 = control-ref of="检测结果"() -> (w341:refnum<vi>)
            n236 = global write "Global.vi" "提示信息"(w344) -> ()
            n237 = global write "Global.vi" "电机结果显示"(w340) -> ()
            n238 = global write "Global.vi" "检测结果"(w341) -> ()
            n239 = global write "Global.vi" "安装支架生产数量"(w342) -> ()
            n240 = global write "Global.vi" "ECU结果显示"(w337) -> ()
            n241 = global write "Global.vi" "电机生产数量"(w338) -> ()
          }
          frame #2 {
            w353 = " " ("值")
            n242 = global read "Global.vi" "ECU结果显示"() -> (w360:refnum<vi>)
            n243 = global read "Global.vi" "电机结果显示"() -> (w362:refnum<vi>)
            n244 = vi-ref "A170316-11_config.vi"() -> (w367:refnum<vi>)
            n245 = control-ref of="ECU装配\n前序状态"() -> (w357:refnum<vi>)
            n246 = control-ref of="电机装配\n前序状态"() -> (w356:refnum<vi>)
            n247 = call "CallVI.vi"("VI引用"=w367, "状态"=T1."Standard") -> ()  [unwired: 11 in, 3 out]
            n248 = global write "Global1.vi" "ECU上序状态"(w357) -> ()
            n249 = global write "Global1.vi" "电机上序状态"(w356) -> ()
            n250 = property class="Str"(reference=w362, "Value"="..." ("结果显示")) -> (reference out=w365:refnum<vi>)  [unwired: 1 in, 1 out]
            n251 = property class="Str"(reference=w360, "Value"="..." ("结果显示")) -> (reference out=w359:refnum<vi>)  [unwired: 1 in, 1 out]
            n252 = property class="Str"(reference=w365, "Text.TextColor"=u32 16776960) -> ()  [unwired: 1 in, 2 out]
            n253 = global read "Global.vi" "电机前序显示字"() -> (w355:refnum<vi>)
            n254 = global read "Global.vi" "ECU前序显示字"() -> (w354:refnum<vi>)
            n255 = property class="Str"(reference=w359, "Text.TextColor"=u32 16776960) -> ()  [unwired: 1 in, 2 out]
            n256 = call "看板状态.vi"("附加信息"="", "设备状态"=enum16{"设备离线", "设备正常", "设备缺料", "设备故障", "质量报警"}."设备正常") -> ("错误输出"=w351:errorcluster)  [unwired: 9 in]
            n257 = disable-structure shown="禁用" {
              frame Disabled {
                n258 = call "看板状态.vi"("附加信息"="", "设备状态"=enum16{"设备离线", "设备正常", "设备缺料", "设备故障", "质量报警"}."设备正常") -> ("错误输出"=w369:errorcluster)  [unwired: 9 in]
              }
              frame Enabled {
              }
            }
            n259 = property class="Str"(reference=w355, "Value"=w353) -> ()  [unwired: 1 in, 2 out]
            n260 = vi-ref "client.vi"() -> (w352:refnum<vi>)
            n261 = property class="Str"(reference=w354, "Value"=w353) -> ()  [unwired: 1 in, 2 out]
            n262 = call "CallVI.vi"("VI引用"=w352, "状态"=T1."Hidden", "错误输入"=w351) -> ()  [unwired: 10 in, 3 out]
            n263 = call "浮动通知.vi"("通知内容"="请选择产品") -> ()  [unwired: 11 in]
          }
        }
        n264 = call <vilib>:"Add State(s) to Queue__jki_lib_state_machine.vi"("State(s) in (\"\")"=w319) -> ("States Out"=w318:string)  [unwired: 14 in]
      }
      frame "UI: Cursor Set" {
        # "Argument"
        n265 = case shown="\"Busy\"" w372 {
          tunnel: w374 -> [w379 w381]
          tunnel: [w378 w380] -> w373
          frame "Idle", Default {
            n266 = call <vilib>:"Unset Busy.vi"("error in (no error)"=w379) -> ("error out"=w378:errorcluster)  [unwired: 10 in]
          }
          frame "Busy" {
            n267 = call <vilib>:"Set Busy.vi"("error in (no error)"=w381) -> ("error out"=w380:errorcluster)  [unwired: 9 in, 1 out]
          }
        }
        n268 = call <vilib>:"Add State(s) to Queue__jki_lib_state_machine.vi"("State(s) in (\"\")"=w377) -> ("States Out"=w376:string)  [unwired: 14 in]
      }
      frame "UI: Front Panel State" {
        # "Argument"
        n269 = Unbundle By Name(w384) -> ("Core.Current VI Reference"=w383:refnum<vi>)
        n270 = case shown="\"Open\", 默认" w382 {
          tunnel: w386 -> [w392 w405]
          tunnel: [w394 w406] -> w385
          tunnel: w383 -> [w393 w403]
          frame "Open", Default {
            n271 = property class="VI"(reference=w393, error in=w392) -> (reference out=w390:refnum<vi>, error out=w391:errorcluster, "Front Panel.Open"=w389:bool)
            n272 = case shown="假" w389 {
              tunnel: [w397 w400] -> w394
              tunnel: w391 -> [w396 w400]
              tunnel: w390 -> [w395 _]
              frame False {
                n273 = invoke class="VI" method="FP.Open"(reference=w395, error in=w396, "Activate"=TRUE, "State"=T1."Standard") -> (error out=w397:errorcluster)  [unwired: 1 in, 4 out]
              }
              frame True {
              }
            }
          }
          frame "Close" {
            n274 = property class="VI"(reference=w403, error in=w405) -> (reference out=w402:refnum<vi>, error out=w404:errorcluster, "Front Panel.Open"=w401:bool)
            n275 = case shown="真" w401 {
              tunnel: [w407 w410] -> w406
              tunnel: w404 -> [w407 w409]
              tunnel: w402 -> [_ w408]
              frame False {
              }
              frame True {
                n276 = invoke class="VI" method="FP.Close"(reference=w408, error in=w409) -> (error out=w410:errorcluster)  [unwired: 1 in, 2 out]
              }
            }
          }
        }
        n277 = call <vilib>:"Add State(s) to Queue__jki_lib_state_machine.vi"("State(s) in (\"\")"=w388) -> ("States Out"=w387:string)  [unwired: 14 in]
      }
      frame "---------- Macro ----------" {
        n278 = call <vilib>:"Add State(s) to Queue__jki_lib_state_machine.vi"("State(s) in (\"\")"=w414) -> ("States Out"=w413:string)  [unwired: 14 in]
      }
      frame "Macro: Initialize" {
        w415 = "Data: Initialize\nInitialize Core Data\nUI: Initialize\nUI: Init\nUI: Front Panel State >> Open"  # Data: Initialize Initialize Core Data UI: Initialize UI: Init UI: Front Panel State >> Open
        n279 = call <vilib>:"Add State(s) to Queue__jki_lib_state_machine.vi"("State(s) in Front (\"\")"=w415, "State(s) in (\"\")"=w419) -> ("States Out"=w418:string)  [unwired: 13 in]
      }
      frame "Macro: Exit" {
        n280 = Unbundle By Name(w431) -> ("Core.Close Panel on Exit?"=w430:bool)
        n281 = vi-ref "client.vi"() -> (w424:refnum<vi>)
        n282 = invoke class="VI" method="Abort VI"(reference=w424) -> (reference out=w423:refnum<vi>, error out=w422:errorcluster)  [unwired: 2 in, 1 out]
        n283 = invoke class="VI" method="FP.Close"(reference=w423, error in=w422) -> (reference out=w421:refnum<vi>, error out=w420:errorcluster)  [unwired: 1 in, 1 out]
        n284 = Select(t="UI: Front Panel State >> Close", s=w430, f="") -> (s? t:f=w427:string)
        n285 = Close Reference(reference=w421, error in (no error)=w420) -> ()  [unwired: 1 out]
        n286 = call <vilib>:"Add State(s) to Queue__jki_lib_state_machine.vi"("State(s) in (\"\")"=w427, "State(s) at Back (\"\")"="Data: Cleanup\nExit") -> ("States Out"=w425:string)  [unwired: 13 in]
        n287 = call <vilib>:"Add State(s) to Queue__jki_lib_state_machine.vi"("State(s) in Front (\"\")"=w425, "State(s) in (\"\")"=w434) -> ("States Out"=w433:string)  [unwired: 13 in]
      }
      frame "---------- New Category ----------" {
        n288 = call <vilib>:"Add State(s) to Queue__jki_lib_state_machine.vi"("State(s) in (\"\")"=w438) -> ("States Out"=w437:string)  [unwired: 14 in]
      }
      frame "New Category: 1" {
        n289 = call <vilib>:"Add State(s) to Queue__jki_lib_state_machine.vi"("State(s) in (\"\")"=w442) -> ("States Out"=w441:string)  [unwired: 14 in]
      }
      frame "New Category: 2" {
        n290 = call <vilib>:"Add State(s) to Queue__jki_lib_state_machine.vi"("State(s) in (\"\")"=w446) -> ("States Out"=w445:string)  [unwired: 14 in]
      }
    }
  }
